vi "transceiverRFID v2.vi"() -> ()   [LabVIEW 2015]
uses:
  <instrlib>/niUSRP/niUSRP Fetch Rx Data (CDB Cluster).vi
  <vilib>/measure/mamon.llb/Trigger Detection for 1 Channel.vi
  <vilib>/Waveform/WDTOps.llb/WDT Get Waveform Subset DBL.vi
  Global_bits.vi
  <instrlib>/niUSRP/niUSRP Write Tx Data (CDB).vi
  <vilib>/measure/NI_MAPro.lvlib
panel:
  out "error out 3":errorcluster
  in  "Parameters Query":T1 {"Session" items=["S0", "S1", "S2", "S3"]; "Sel" items=["All", "All2", "~SL", "SL"]; "M" items=["M=1", "M=2", "M=4", "M=8"]}
  in  "Symbol Rate [Hz]":dbl=500000.0 format="%#_13p"
  in  "Parameters Select":T2={"Target"=7, "Action"=0, "MemBank"=1, "truncate"=FALSE} {"MemBank" items=["00 RFU", "01 EPC", "10 TID", "11 User"]; "Action" items=["000", "001", "010", "011", "100", "101", "110", "111"]; "Target" items=["000 Inventoried (S0)", "001 Inventoried (S1)", "010 Inventoried (S2)", "011 Inventoried (S3)", "100 SL", "101 RFU", "110 RFU", "111 RFU"]}
  in  "Parameters Symbols":T3={"Tari"=8e-06, "PW"=0.5, "factor for \"1\" symbol"=0.5, "RTcal"=2.5, "TRcal"=3.0, "Delimiter"=1.4e-05} {"TRcal" min=1.1 max=3.0 step=0.1; "RTcal" min=2.5 max=3.0 step=0.1; "factor for \"1\" symbol" min=0.5 max=1.0 step=0.1; "PW" min=0.265 max=0.525 step=0.001; "Tari" format="%#_3p"}
  out "coerced IQ rate 2":dbl=100000.0 format="%#_6p"
  out "carrier frequency 3":dbl=100000.0 format="%#_6p"
  out "coerced gain 2":dbl format="%#_6f"
  in  "stop":bool
  out "Loop":i32
  out "RFID Pushed":bool
  in  "query":bool
  out "RN16 array":i32[](array[numeric])=[0, 1, 1, 0, 0, 0, 1, 0, 1, 1, 1, 1, 1, 1, 1, 1]
  out "bits":i16[](graph)=[1, 1, 1, 1, 0, 0, 1, 0, 0, 0, 1, 1, 0, 0, 0, 0, 0, 1, 1, 1, 0, 0, 1, 0, 0, 0, 0, 1, 1, 1, 0, 0, 1, 0, 0, 1, 0, 0, 1, 0, 0, 0, 0, 1, 1, 0, 1, 1, 1, 0, 0, 0, 0, 1, 1, 1, 0, 0, 0, 1, 1, 1, 0, 0, 0, 0, 1, 1, 1, 0, 0, 0, 0, 1, 1, 1, 0, 0, 0, 0, 0, 0, 0, 0]
  out "Wave Mag":dbl[](graph)
  out "ACK":bool
  in  "IQ rate 2":dbl=2000000.0 format="%#_6p"
  in  "carrier frequency 2":dbl=920000000.0 format="%#_6p"
  in  "gain 2":dbl format="%#_6f"
  in  "tx device names":refnum<k15>="192.168.20.13"
  in  "active antenna":string="RX2"
  in  "Channels":string(combo)="0"
  in  "timeout":dbl=10.0
  in  "number of samples":i64=2000000
  in  "Stop":bool
  out "Magnitude":cluster{"t0":dbl, "dt":dbl, "Y":dbl[]}(graph)={"t0"=425.94010384, "dt"=5e-07, "Y"=array[2000000 elements]}
  out "Triggered Signal":dynamicdata(graph)=[{"t0"=timestamp(16448802 s since 1904-01-01), "dt"=1.0, "Y"=array[750 elements], "attributes"=variant("NI_ChannelName"=variant(string "Trigger"))}]
  out "Portion Signal":dynamicdata(graph)=[{"t0"=timestamp(3606796793.4692063 s since 1904-01-01), "dt"=1.0, "Y"=[0.175, 0.175, 0.175, 0.175, 0.215, 0.215, 0.215, 0.175, 0.175, 0.215, 0.215, 0.175, 0.175, 0.175, 0.215, 0.215, 0.175, 0.215, 0.215, 0.175, 0.175, 0.215, 0.175, 0.175, 0.215, 0.215, 0.175, 0.215, 0.215, 0.175, 0.175, 0.215, 0.175, 0.175, 0.215, 0.175, 0.175, 0.215, 0.215, 0.175, 0.215, 0.215, 0.175, 0.175, 0.215, 0.175, 0.175, 0.215, 0.175, 0.175, 0.215, 0.215, 0.175, 0.175, 0.215, 0.175, 0.175, 0.215, 0.175, 0.175, 0.215, 0.215, 0.215, 0.175, 0.175, 0.215, 0.175, 0.175, 0.175, 0.175, 0.215, 0.215, 0.215, 0.175, 0.175, 0.215, 0.175, 0.175, 0.215, 0.175, 0.175, 0.215, 0.215, 0.175, 0.175, 0.215, 0.175, 0.175, 0.215, 0.175, 0.175, 0.215, 0.175, 0.175, 0.215, 0.215, 0.175, 0.175, 0.215, 0.175, 0.175, 0.215, 0.175, 0.175, 0.215, 0.215, 0.175, 0.175, 0.215, 0.175, 0.175, 0.215, 0.175, 0.175, 0.215, 0.215, 0.175, 0.215, 0.215, 0.175, 0.175, 0.215, 0.175, 0.175, 0.215, 0.175, 0.175, 0.215, 0.215, 0.175, 0.175, 0.215, 0.175, 0.175, 0.215, 0.175, 0.175, 0.215, 0.175, 0.175, 0.215, 0.215, 0.175, 0.175, 0.215, 0.175, 0.175, 0.215, 0.175, 0.175, 0.215, 0.215, 0.175, 0.175, 0.215, 0.175, 0.175, 0.215, 0.175, 0.175, 0.215, 0.175, 0.175, 0.215, 0.215, 0.175, 0.175, 0.215, 0.175, 0.175, 0.215, 0.175, 0.175, 0.215, 0.175, 0.175, 0.215, 0.215, 0.175, 0.175]}, {"t0"=timestamp(16449352 s since 1904-01-01), "dt"=1.0, "Y"=[0.6542204406555878, 0.6330066792866885, 0.6289206010452267, 0.626525788591559, 0.6440170826344898, 0.6558913247662658, 0.6551466050382949, 0.6446576873057327, 0.6276789703693967, 0.6487660336682352, 0.6515045603831945, 0.6315654455000962, 0.6285598365750038, 0.6291977552419075, 0.6513744582179881, 0.6487718708937794, 0.6281161281271066, 0.6441036383531251, 0.6540546398928915, 0.6323048994250363, 0.6359679052689398, 0.6558585780757112, 0.6396687990551979, 0.629156140414305, 0.6518867729873677, 0.6483523017326835, 0.6287998621524823, 0.6479419819057154, 0.6523620464006552, 0.6302348513521957, 0.6394592548080206, 0.6560056754287461, 0.6353038672852097, 0.6346389862773866, 0.6557564358134849, 0.6402277966255374, 0.6287483168841594, 0.651006297610194, 0.6487867644817977, 0.6294605495842085, 0.6476222426699878, 0.652197032759818, 0.6297422152107712, 0.638725861964971, 0.6556999088508416, 0.6357702096227417, 0.6303899874831843, 0.6536513023112432, 0.6453874681954346, 0.6282678144317502, 0.6470302178597716, 0.6522701409900283, 0.6299221874750973, 0.642426414545514, 0.6547052180570018, 0.6323249481039205, 0.6333552552398422, 0.6553467581989884, 0.6405086905627353, 0.6315662027705019, 0.6526133380528634, 0.6535557019281786, 0.654421911761707, 0.6380373636097645, 0.6307874460100164, 0.6536176318748712, 0.6406224634572578, 0.6270835009019179, 0.6269903627063104, 0.6338698329632815, 0.6536116384280213, 0.653257077985277, 0.6533937223519337, 0.6338942026134534, 0.6331043491528318, 0.6547473769267388, 0.6411190331089638, 0.6275601609203197, 0.6496280391371777, 0.6458061649598519, 0.6267659422503373, 0.6452588001110147, 0.6524795072180846, 0.6299948003589266, 0.6366571347752407, 0.6536005142113043, 0.632409054009175, 0.6318732943523131, 0.6539270504909295, 0.6414501140307582, 0.6276388315395326, 0.6491703842752117, 0.6458834206984477, 0.6262937266147462, 0.6443153980416729, 0.6519924520978075, 0.629042357653491, 0.6353287837179523, 0.6545296689316882, 0.6369081613804035, 0.6290638058284929, 0.6512822332544489, 0.6457777456866854, 0.6263645066376707, 0.6442292350994769, 0.6496124314718684, 0.6268011308873612, 0.6393831799145786, 0.6540143802735646, 0.633088873311549, 0.6314470575578446, 0.6529060917394062, 0.6369507583109556, 0.6280382313641445, 0.6507502705684688, 0.6457390376488532, 0.6257248776510101, 0.6436289616350072, 0.6499581940450706, 0.6274609957119216, 0.6388504902100247, 0.6536636816864714, 0.6331735786644757, 0.6306605221497352, 0.652740208254182, 0.64128117204542, 0.6258860788907208, 0.6468182432467872, 0.6496205615265724, 0.6272331501727273, 0.6382326153017709, 0.6518270541144702, 0.629643965384008, 0.6335678245703787, 0.6533675162201217, 0.6366936469982558, 0.6262540961233908, 0.6495447267673374, 0.6419769674391187, 0.6253642504421832, 0.6456429465893609, 0.6490760180330309, 0.6268146564515095, 0.6374754890127863, 0.6517341322079381, 0.6289016397242593, 0.6323826159966556, 0.6531167564613976, 0.637130944131767, 0.626625252663772, 0.6488663115123084, 0.6458866479589179, 0.6257091686813125, 0.6408464802006677, 0.6515973320665904, 0.628676080037199, 0.6319590623959827, 0.652097765579169, 0.633324553683118, 0.6285426588530133, 0.6505853921308588, 0.6415519048673486, 0.6245075306846388, 0.6447252096283556, 0.6459387707408372, 0.6241539664908139, 0.6401210700943205, 0.6516950719440161, 0.6296678507097518, 0.6316662953086386, 0.6517458063157089, 0.6333743530720075, 0.627704200597501, 0.6504285603489174, 0.6412976730640289, 0.6238942612116077, 0.6437532229968528, 0.649057237990462, 0.6263972072140956, 0.6345010038828095], "attributes"=variant("NI_ChannelName"=variant(string "Trigger"))}]
  out "start samples":dbl format="%.3g"
  out "duration samples":dbl format="%.3g"
  in  "start":i64=550 format="%.3g"
  in  "duration":dbl=180.0 format="%#_13g"
  out "RN16 waveform":i16[](graph)
  out "error out 2":errorcluster
  out "loop":i32
  out "trigger location":dbl format="%#_2g"
  out "Trigger":bool
  out "coerced gain":dbl format="%#_6f"
  out "coerced carrier frequency":dbl=100000.0 format="%#_6p"
  out "coerced IQ rate":dbl=100000.0 format="%#_6p"
  in  "gain":dbl format="%#_6f"
  in  "carrier frequency":dbl=920000000.0 format="%#_6p"
  in  "IQ rate":dbl=2000000.0 format="%#_6p"
  out "error out":errorcluster
  in  "device names":refnum<k15>="192.168.10.14"
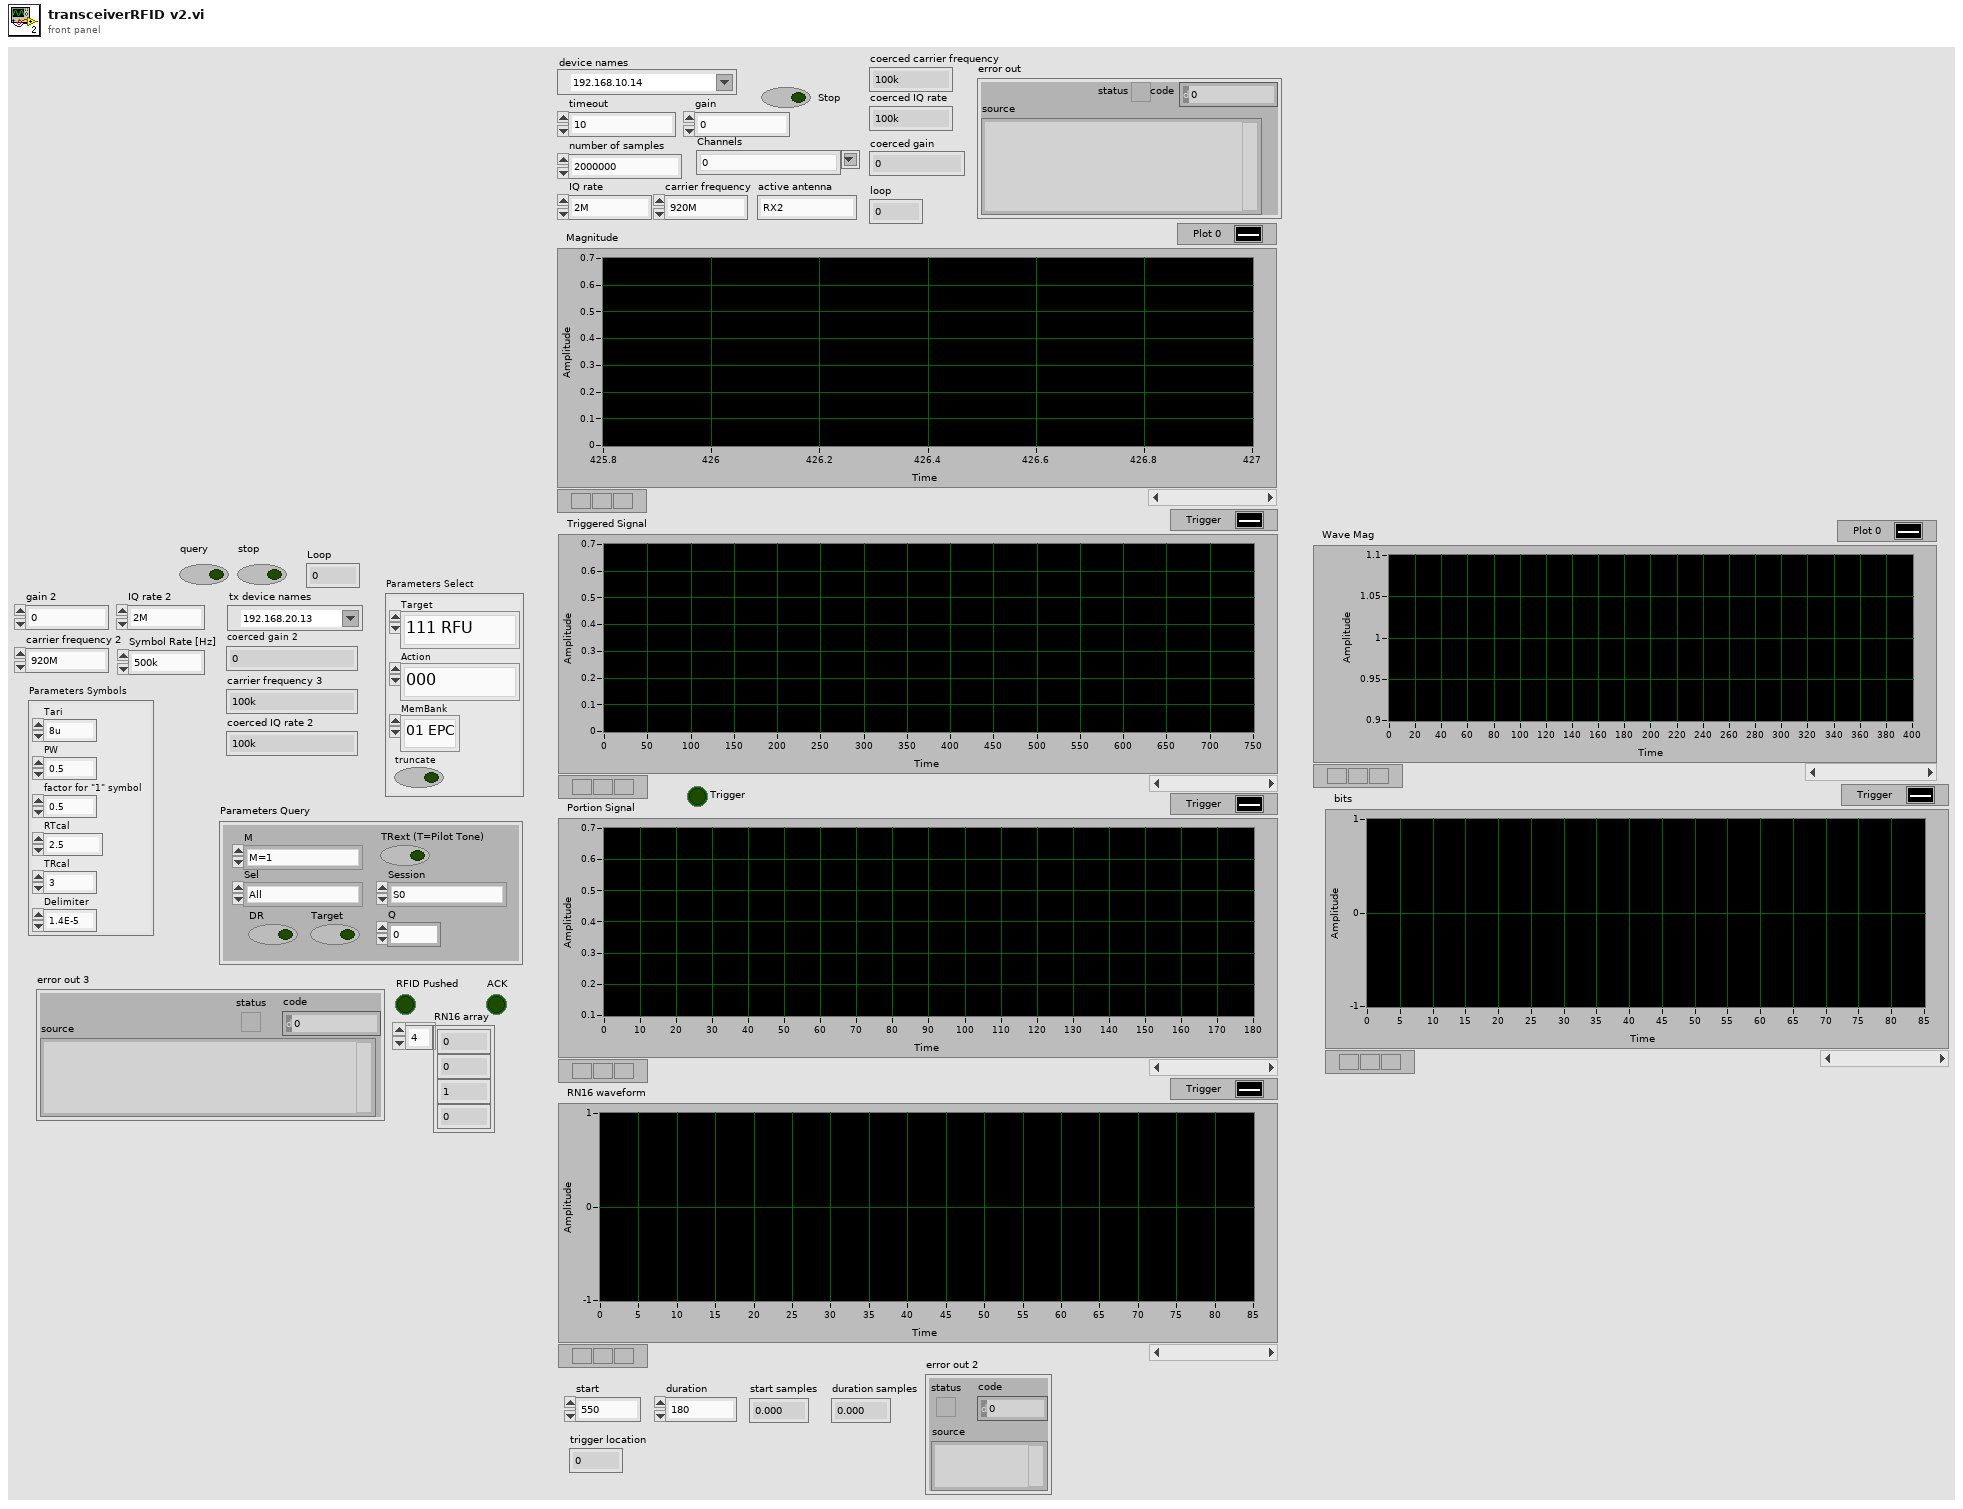
[diagram p1: front panel]
types:
  T1 = cluster{"DR":bool, "M":u16, "TRext (T=Pilot Tone)":bool, "Sel":u16, "Session":u16, "Q":u8, "Target":bool}
  T2 = cluster{"Target":u16, "Action":u16, "MemBank":u16, "truncate":bool}
  T3 = cluster{"Tari":dbl, "PW":dbl, "factor for \"1\" symbol":dbl, "RTcal":dbl, "TRcal":dbl, "Delimiter":dbl}
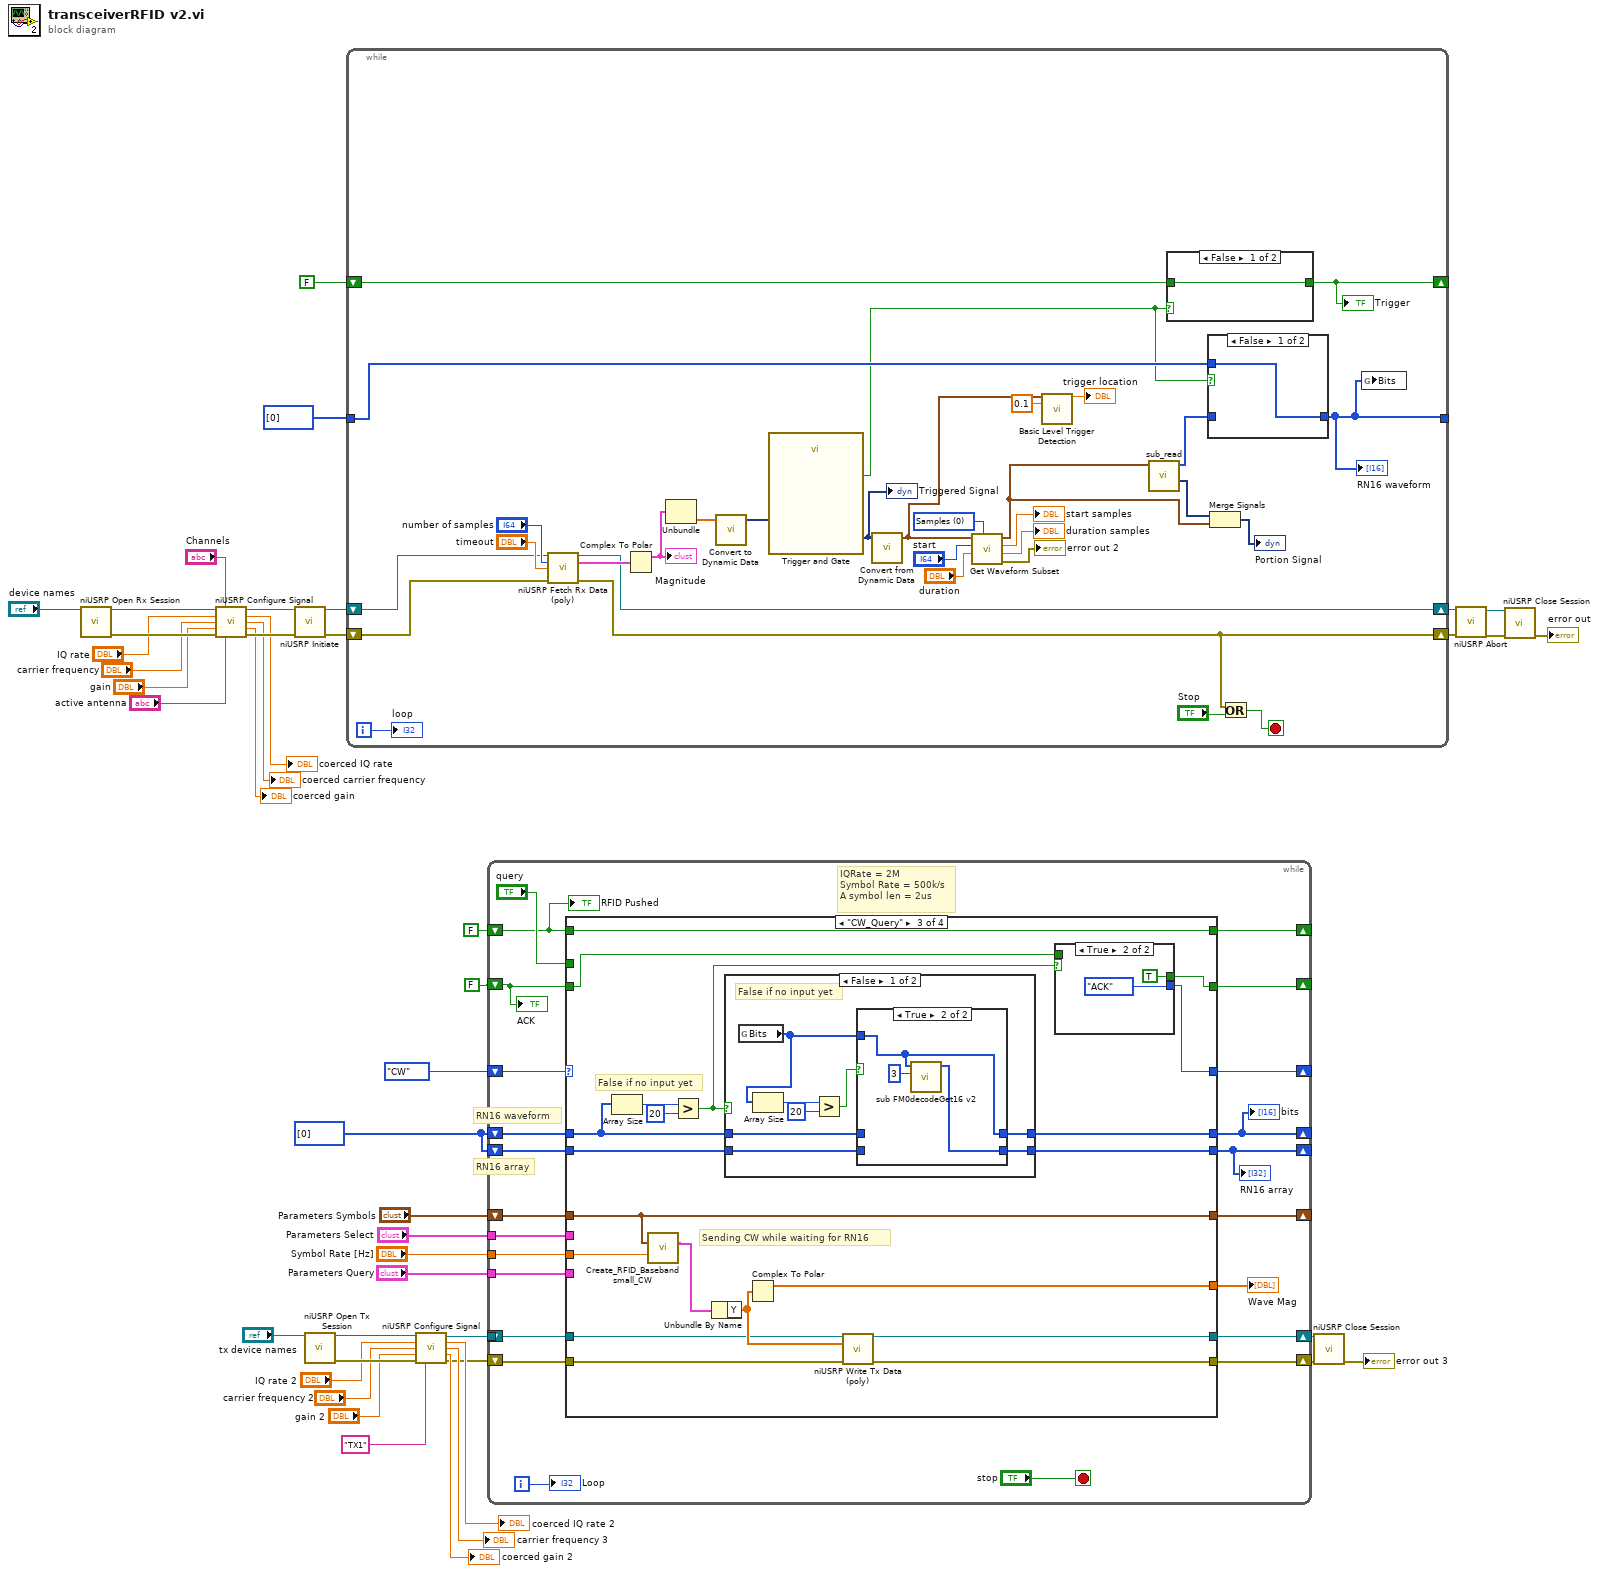
[diagram p0: block diagram]
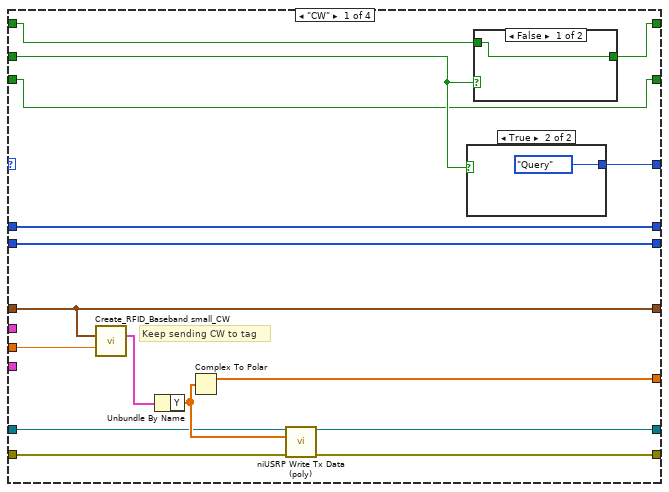
[diagram p2: hidden frame]
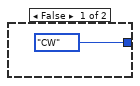
[diagram p4: hidden frame]
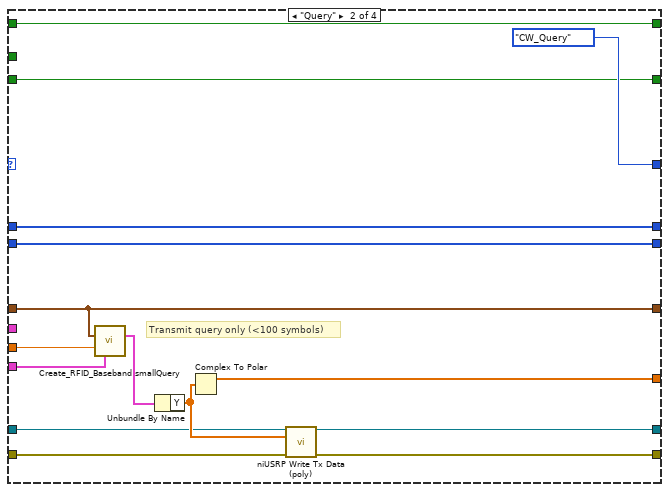
[diagram p5: hidden frame]
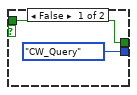
[diagram p6: hidden frame]
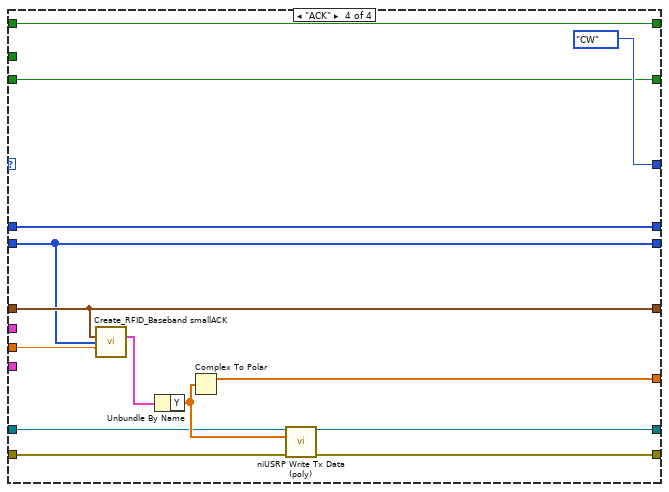
[diagram p9: hidden frame]
diagram:
  w1 = i16[] [0]
  # "RN16 array"
  # "RN16 waveform"
  n1 = call <instrlib>:"niUSRP Open Rx Session.vi"("device names"="device names") -> ("session handle out"=w44:refnum<k15>, "error out"=w43:errorcluster)  [unwired: 13 in]
  n2 = call <instrlib>:"niUSRP Configure Signal.vi"("session handle"=w44, "channel list"="Channels", "IQ rate"="IQ rate", "carrier frequency"="carrier frequency", "gain"="gain", "error in (no error)"=w43, "active antenna"="active antenna") -> ("session handle out"=w42:refnum<k15>, "coerced IQ rate"=→"coerced IQ rate":dbl, "coerced carrier frequency"=→"coerced carrier frequency":dbl, "coerced gain"=→"coerced gain":dbl, "error out"=w41:errorcluster)  [unwired: 4 in]
  n3 = call <instrlib>:"niUSRP Initiate.vi"("session handle"=w42, "error in (no error)"=w41) -> ("session handle out"=w40:refnum<k15>, "error out"=w39:errorcluster)  [unwired: 12 in]
  n4 = call <instrlib>:"niUSRP Open Tx Session.vi"("device names"="tx device names") -> ("session handle out"=w4:refnum<k15>, "error out"=w23:errorcluster)  [unwired: 13 in]
  n5 = while {
    shift-right: [w74] -> w38
    shift-left: w40 -> [w73]
    shift-right: [w57] -> w37
    shift-left: w39 -> [w72]
    shift-right: [w50] -> _
    shift-left: FALSE -> [w49]
    tunnel: i16[] [0] -> [w54]
    tunnel: [w46] -> _
    i -> [w56]
    stop <- w69 stop-if-true
    w66 = u16 0 items=["Samples", "Relative Time"] ("start/duration format")
    n6 = call-poly <instrlib>:"niUSRP Fetch Rx Data (poly).vi"("session handle"=w73, "number of samples"="number of samples", "timeout"="timeout", "error in (no error)"=w72) -> ("session handle out"=w74:refnum<k15>, "data"=w75:cluster{"t0":dbl, "dt":dbl, "Y":cdb[]}, "error out"=w57:errorcluster)  [unwired: 8 in, 1 out]
    n7 = Complex To Polar(r * e^(i*theta)=w75) -> (r=w71:cluster{"t0":dbl, "dt":dbl, "Y":dbl[]})  [unwired: 1 out]
    "Magnitude" <- w71
    n8 = Unbundle(w71) -> ("Y"=w60:dbl[])  [unwired: 2 out]
    n9 = call "Convert to Dynamic Data"("Array"=w60) -> ("Dynamic Data Type"=w70:dynamicdata)  [unwired: 3 in]
    n10 = call "Trigger and Gate"("Signals"=w70) -> ("Triggered Signals"=w63:dynamicdata, "Data Available"=w48:bool)  [unwired: 7 in, 2 out]
    "Triggered Signal" <- w63
    n11 = call "Convert from Dynamic Data"("Dynamic Data Type"=w63) -> ("Waveform"=w51:waveform(dbl))  [unwired: 3 in]
    n12 = call-poly <vilib>:"Get Waveform Subset.vi"("start/duration format"=w66, "duration"="duration", "start samples/time"="start", "waveform in"=w51) -> ("error out"=→"error out 2":errorcluster, "actual duration"=→"duration samples":dbl, "actual start samples/time"=→"start samples":dbl, "waveform out"=w53:waveform(dbl))  [unwired: 2 in]
    n13 = call-poly <vilib>:"Basic Level Trigger Detection.vi"("signal in"=w51, "level"=0.1) -> ("trigger location"=→"trigger location":dbl)  [unwired: 11 in, 2 out]
    n14 = call "sub_read.vi"("Raw Signal"=w53) -> ("Digitized Sign"=w62:dynamicdata, "Bits"=w55:i16[])  [unwired: 6 in, 2 out]
    n15 = case shown="False" w48 {
      selector: w48 -> [_ w79]
      tunnel: [w78 w79] -> w50
      tunnel: w49 -> [w78 _]
      frame False {
      }
      frame True {
      }
    }
    "Trigger" <- w50
    n16 = case shown="False" w48 {
      tunnel: w55 -> [_ w81]
      tunnel: [w80 w81] -> w46
      tunnel: w54 -> [w80 _]
      frame False {
      }
      frame True {
      }
    }
    "RN16 waveform" <- w46
    n17 = Merge Signals(w62, w53) -> (→"Portion Signal":dynamicdata)
    n18 = Or(x=w57, y="Stop") -> (x .or. y?=w69:bool)
    n19 = global write "Global_bits.vi" "Bits"(w46) -> ()
    "loop" <- w56
  }
  n20 = call <instrlib>:"niUSRP Configure Signal.vi"("session handle"=w4, "IQ rate"="IQ rate 2", "carrier frequency"="carrier frequency 2", "gain"="gain 2", "error in (no error)"=w23, "active antenna"="TX1") -> ("session handle out"=w10:refnum<k15>, "coerced IQ rate"=→"coerced IQ rate 2":dbl, "coerced carrier frequency"=→"carrier frequency 3":dbl, "coerced gain"=→"coerced gain 2":dbl, "error out"=w9:errorcluster)  [unwired: 5 in]
  n21 = while {
    tunnel: "Parameters Select" -> [w97]
    tunnel: "Parameters Query" -> [w95]
    tunnel: w10 -> [w102]
    shift-right: [w100] -> w8
    shift-left: w9 -> [w101]
    shift-right: [w99] -> w6
    shift-left: _ -> [_]
    shift-right: [w92] -> _
    shift-left: enum16{"CW", "Query", "CW_Query", "ACK"}."CW" -> [w103]
    shift-right: [w94] -> _
    shift-left: "Parameters Symbols" -> [w98]
    tunnel: "Symbol Rate [Hz]" -> [w96]
    shift-right: [w90] -> _
    shift-left: w1 -> [w91]
    shift-right: [w89] -> _
    shift-left: w1 -> [w88]
    shift-right: [w85] -> _
    shift-left: FALSE ("query") -> [w84]
    shift-right: [w82] -> _
    shift-left: FALSE ("query") -> [w83]
    i -> [w104]
    stop <- "stop" stop-if-true
    # "IQRate = 2M\nSymbol Rate = 500k/s\nA symbol len = 2us"
    n22 = case shown="\"CW_Query\"" w103 {
      tunnel: w102 -> [w119 w138 w158 w191]
      tunnel: w101 -> [w118 w137 w157 w190]
      tunnel: [w117 w136 w156 w189] -> w100
      tunnel: [w116 w135 w155 w188] -> w99
      tunnel: w98 -> [w114 w130 w146 w186]
      tunnel: w97 -> [_ _ _ _]
      tunnel: w96 -> [w113 w131 w145 w185]
      tunnel: w95 -> [_ w132 _ _]
      tunnel: [w114 w130 w146 w186] -> w94
      tunnel: [w115 w134 w154 w187] -> w87
      tunnel: [w111 enum16{"CW", "Query", "CW_Query", "ACK"}."CW_Query" w143 enum16{"CW", "Query", "CW_Query", "ACK"}."CW"] -> w92
      tunnel: "query" -> [w108 _ _ _]
      tunnel: w91 -> [w110 w129 w151 w182]
      tunnel: [w110 w129 w149 w182] -> w90
      tunnel: [w109 w128 w150 w183] -> w89
      tunnel: w88 -> [w109 w128 w148 w183]
      tunnel: [w107 w126 w142 w180] -> w85
      tunnel: w84 -> [w106 w126 w142 w180]
      tunnel: w83 -> [w105 w125 w141 w179]
      tunnel: [w105 w125 w140 w179] -> w82
      frame "CW" {
        # "Keep sending CW to tag"
        n23 = call "Create_RFID_Baseband small_CW.vi"("Parameters Symbols"=w114, "Symbol Rate [Hz]"=w113) -> ("complex waveform"=w112:cluster{"t0":dbl, "dt":dbl, "Y":cdb[]})  [unwired: 12 in, 1 out]
        n24 = Unbundle By Name(w112) -> ("Y"=w120:cdb[])
        n25 = Complex To Polar(r * e^(i*theta)=w120) -> (r=w115:dbl[])  [unwired: 1 out]
        n26 = call-poly <instrlib>:"niUSRP Write Tx Data (poly).vi"("session handle"=w119, "data"=w120, "error in (no error)"=w118) -> ("session handle out"=w116:refnum<k15>, "error out"=w117:errorcluster)  [unwired: 11 in]
        n27 = case shown="True" w108 {
          tunnel: [enum16{"CW", "Query", "CW_Query", "ACK"}."CW" enum16{"CW", "Query", "CW_Query", "ACK"}."Query"] -> w111
          frame False {
          }
          frame True {
          }
        }
        n28 = case shown="False" w108 {
          selector: w108 -> [_ w122]
          tunnel: [w121 w122] -> w107
          tunnel: w106 -> [w121 _]
          frame False {
          }
          frame True {
          }
        }
      }
      frame "Query" {
        # "Transmit query only (<100 symbols)"
        n29 = call "Create_RFID_Baseband smallQuery.vi"("Parameters Symbols"=w130, "Symbol Rate [Hz]"=w131, "Parameters Query"=w132) -> ("complex waveform"=w133:cluster{"t0":dbl, "dt":dbl, "Y":cdb[]})  [unwired: 11 in, 1 out]
        n30 = Unbundle By Name(w133) -> ("Y"=w139:cdb[])
        n31 = Complex To Polar(r * e^(i*theta)=w139) -> (r=w134:dbl[])  [unwired: 1 out]
        n32 = call-poly <instrlib>:"niUSRP Write Tx Data (poly).vi"("session handle"=w138, "data"=w139, "error in (no error)"=w137) -> ("session handle out"=w135:refnum<k15>, "error out"=w136:errorcluster)  [unwired: 11 in]
      }
      frame "CW_Query" {
        # "False if no input yet"
        # "Sending CW while waiting for RN16"
        n33 = Array Size(array=w151) -> (size(s)=w152:i32)
        n34 = call "Create_RFID_Baseband small_CW.vi"("Parameters Symbols"=w146, "Symbol Rate [Hz]"=w145) -> ("complex waveform"=w147:cluster{"t0":dbl, "dt":dbl, "Y":cdb[]})  [unwired: 12 in, 1 out]
        n35 = Greater?(x=w152, y=20) -> (0:w144:bool)
        n36 = Unbundle By Name(w147) -> ("Y"=w159:cdb[])
        n37 = case shown="False" w144 {
          tunnel: [w168 w178] -> w149
          tunnel: w151 -> [w165 w178]
          tunnel: [w167 w177] -> w150
          tunnel: w148 -> [w166 w177]
          frame False {
            # "False if no input yet"
            n38 = global read "Global_bits.vi" "Bits"() -> (w164:i16[])
            n39 = Array Size(array=w164) -> (size(s)=w171:i32)
            n40 = Greater?(x=w171, y=20) -> (0:w169:bool)
            n41 = case shown="True" w169 {
              tunnel: w165 -> [w173 _]
              tunnel: [w173 w174] -> w168
              tunnel: [w172 w176] -> w167
              tunnel: w166 -> [w172 _]
              tunnel: w164 -> [_ w174]
              frame False {
              }
              frame True {
                n42 = call "sub FM0decodeGet16 v2.vi"("threshold"=3, "RN16 waveform"=w174) -> ("RN16 array"=w176:i32[])  [unwired: 9 in]
              }
            }
          }
          frame True {
          }
        }
        n43 = Complex To Polar(r * e^(i*theta)=w159) -> (r=w154:dbl[])  [unwired: 1 out]
        n44 = call-poly <instrlib>:"niUSRP Write Tx Data (poly).vi"("session handle"=w158, "data"=w159, "error in (no error)"=w157) -> ("session handle out"=w155:refnum<k15>, "error out"=w156:errorcluster)  [unwired: 11 in]
        n45 = case shown="True" w144 {
          tunnel: [enum16{"CW", "Query", "CW_Query", "ACK"}."CW_Query" enum16{"CW", "Query", "CW_Query", "ACK"}."ACK"] -> w143
          tunnel: w141 -> [w160 _]
          tunnel: [w160 TRUE ("query")] -> w140
          frame False {
          }
          frame True {
          }
        }
      }
      frame "ACK" {
        n46 = call "Create_RFID_Baseband smallACK.vi"("Parameters Symbols"=w186, "RN16 array"=w183, "Symbol Rate [Hz]"=w185) -> ("complex waveform"=w184:cluster{"t0":dbl, "dt":dbl, "Y":cdb[]})  [unwired: 11 in, 1 out]
        n47 = Unbundle By Name(w184) -> ("Y"=w192:cdb[])
        n48 = Complex To Polar(r * e^(i*theta)=w192) -> (r=w187:dbl[])  [unwired: 1 out]
        n49 = call-poly <instrlib>:"niUSRP Write Tx Data (poly).vi"("session handle"=w191, "data"=w192, "error in (no error)"=w190) -> ("session handle out"=w188:refnum<k15>, "error out"=w189:errorcluster)  [unwired: 11 in]
      }
    }
    "RN16 array" <- w89
    "bits" <- w90
    "Wave Mag" <- w87
    "Loop" <- w104
    "RFID Pushed" <- w84
    "ACK" <- w83
  }
  n50 = call <instrlib>:"niUSRP Close Session.vi"("session handle"=w6, "error in (no error)"=w8) -> ("error out"=→"error out 3":errorcluster)  [unwired: 13 in]
  n51 = call <instrlib>:"niUSRP Abort.vi"("session handle"=w38, "error in (no error)"=w37) -> ("session handle out"=w36:refnum<k15>, "error out"=w35:errorcluster)  [unwired: 12 in]
  n52 = call <instrlib>:"niUSRP Close Session.vi"("session handle"=w36, "error in (no error)"=w35) -> ("error out"=→"error out":errorcluster)  [unwired: 13 in]
